vi "HFRR ADV v037.vi"() -> ()   [LabVIEW 2025] (continued)
        n1323 = Not(x=w1614) -> (.not. x?=w1612:bool)
        n1324 = local write "Stroke"(w1612) -> ()
        n1325 = local write "Tab Control 2"(T6."Stroke" ("Tab Control 2")) -> ()
      }
    }
    n1326 = local write "tested by"(w1341) -> ()
    n1327 = case shown="True" w1337 {
      selector: w1337 -> [_ w1617]
      frame False {
      }
      frame True {
        n1328 = Not(x=w1617) -> (.not. x?=w1615:bool)
        n1329 = local write "Humidity"(w1615) -> ()
        n1330 = local write "Tab Control 2"(T6."Humidity" ("Tab Control 2")) -> ()
      }
    }
    n1331 = case shown="\"Calibration\"" "Main Dashboard Buttons" {
      tunnel: [T2."HOME" ("Main Tab") T2."Test Setup" ("Main Tab") T2."Acquire" ("Main Tab") T2."Adv Scar" ("Main Tab") T2."Adv Scar Report" ("Main Tab") T2."Compare Files" ("Main Tab") T2."Calibration" ("Main Tab") T2."About" ("Main Tab") T2."Advance" ("Main Tab")] -> w1320
      frame "Home", Default {
      }
      frame "Test Setup" {
      }
      frame "Dashboard" {
      }
      frame "Imaging" {
      }
      frame "Report" {
      }
      frame "Analysis" {
      }
      frame "Calibration" {
      }
      frame "About" {
      }
      frame "Advance" {
      }
    }
    n1332 = Wait (ms)(milliseconds to wait=u32 100) -> ()  [unwired: 1 out]
    n1333 = local read "Main Tab Display"() -> (w1340:T4)
    n1334 = local write "Main Tab"(w1320) -> ()
    n1335 = case shown="\"Dashboard 3\"" w1340 {
      frame "Dashboard 1", Default {
        n1336 = property on="Reset Graph" class="Bool (strict)"("Visible"=FALSE) -> ()  [unwired: 2 in, 2 out]
      }
      frame "Dashboard 2" {
        n1337 = property on="Reset Graph" class="Bool (strict)"("Visible"=TRUE) -> ()  [unwired: 2 in, 2 out]
      }
      frame "Dashboard 3" {
        n1338 = property on="Reset Graph" class="Bool (strict)"("Visible"=TRUE) -> ()  [unwired: 2 in, 2 out]
      }
    }
    n1339 = local read "SCAR MEASURMENT"() -> (w1328:enum32{"Auto Scar", "Manual Scar"})
    n1340 = local read "Humidity"() -> (w1342:bool)
    n1341 = local read "Cap Live Image"() -> (w1325:bool)
    n1342 = local read "Sample Temperature"() -> (w1335:bool)
    n1343 = local read "Air Temp vs Humidity"() -> (w1333:bool)
    n1344 = local read "Frequency"() -> (w1334:bool)
    n1345 = case shown="False" w1342 {
      frame False {
        n1346 = local write "Humidity On Command"(TRUE ("Humidity On Command")) -> ()
        n1347 = case shown="True" "Humidity Off Command" {
          selector: "Humidity Off Command" -> [_ w1630]
          frame False {
          }
          frame True {
            n1348 = stacked-sequence {
              frame #0 {
                n1349 = local read "WriteHumidity"() -> (w1632:string[])
                n1350 = Insert Into Array(array=w1632, new element="R;1" ("new element/subarray")) -> (w1631:string[])  [unwired: 1 in]
                n1351 = local write "WriteHumidity"(w1631) -> ()
              }
              frame #1 {
                n1352 = Wait (ms)(milliseconds to wait=u32 500) -> ()  [unwired: 1 out]
              }
              frame #2 {
                n1353 = local read "WriteHumidity"() -> (w1636:string[])
                n1354 = local read "EVENT LOG"() -> (w1640:string)
                n1355 = call "Event Log.vi"("Content"="Humidity Control Off" ("string"), "EVENT LOG"=w1640) -> ("EVENT LOG"=w1641:string)  [unwired: 8 in, 1 out]
                n1356 = local write "EVENT LOG"(w1641) -> ()
                n1357 = Insert Into Array(array=w1636, new element="R;1" ("new element/subarray")) -> (w1637:string[])  [unwired: 1 in]
                n1358 = local write "WriteHumidity"(w1637) -> ()
                n1359 = local write "Humidity"(TRUE ("Humidity")) -> ()
              }
            }
            n1360 = Not(x=w1630) -> (.not. x?=w1629:bool)
            n1361 = local write "Humidity Off Command"(w1629) -> ()
          }
        }
      }
      frame True {
        n1362 = local write "Humidity Off Command"(TRUE ("Humidity Off Command")) -> ()
        n1363 = case shown="False" "Humidity On Command" {
          selector: "Humidity On Command" -> [_ w1645]
          frame False {
          }
          frame True {
            n1364 = stacked-sequence {
              frame #0 {
                n1365 = local read "Set Rh"() -> (w1651:dbl)
                n1366 = local read "WriteHumidity"() -> (w1647:string[])
                n1367 = Number To Fractional String(number=w1651, precision (6)=i16 2) -> (F-format string=w1652:string)  [unwired: 2 in]
                n1368 = Concatenate Strings("M;" ("new element/subarray"), w1652) -> (w1650:string)
                n1369 = Insert Into Array(array=w1647, new element=w1650) -> (w1646:string[])  [unwired: 1 in]
                n1370 = local write "WriteHumidity"(w1646) -> ()
              }
              frame #1 {
                n1371 = Wait (ms)(milliseconds to wait=u32 500) -> ()  [unwired: 1 out]
              }
              frame #2 {
                n1372 = local read "WriteHumidity"() -> (w1655:string[])
                n1373 = local read "Set Rh"() -> (w1659:dbl)
                n1374 = Number To Fractional String(number=w1659, precision (6)=i16 2) -> (F-format string=w1660:string)  [unwired: 2 in]
                n1375 = Concatenate Strings("M;" ("new element/subarray"), w1660) -> (w1658:string)
                n1376 = Insert Into Array(array=w1655, new element=w1658) -> (w1654:string[])  [unwired: 1 in]
                n1377 = local write "WriteHumidity"(w1654) -> ()
              }
              frame #3 {
                n1378 = Wait (ms)(milliseconds to wait=u32 500) -> ()  [unwired: 1 out]
              }
              frame #4 {
                (unwired) "% RH" ("string")
                (unwired) i16 2 ("precision (6)")
                (unwired) "M;" ("new element/subarray")
                n1379 = local read "Set Rh"() -> (w1669:dbl)
                n1380 = local read "WriteHumidity"() -> (w1662:string[])
                n1381 = Number To Fractional String(number=w1669, precision (6)=i16 2) -> (F-format string=w1666:string)  [unwired: 2 in]
                n1382 = Concatenate Strings("M;" ("new element/subarray"), w1666) -> (w1670:string)
                n1383 = Concatenate Strings("Humidity Set to : " ("string"), w1666, "% RH" ("string")) -> (w1664:string)
                n1384 = Insert Into Array(array=w1662, new element=w1670) -> (w1663:string[])  [unwired: 1 in]
                n1385 = disable-structure shown="Enabled" {
                  frame Enabled {
                    n1386 = local read "EVENT LOG"() -> (w1673:string)
                    n1387 = call "Event Log.vi"("Content"="Humidity Control On", "EVENT LOG"=w1673) -> ("EVENT LOG"=w1674:string)  [unwired: 8 in, 1 out]
                    n1388 = local write "EVENT LOG"(w1674) -> ()
                  }
                  frame Disabled {
                  }
                }
                n1389 = disable-structure shown="Enabled" {
                  disable-tunnel: w1664 -> [_ _]
                  frame Enabled {
                    n1390 = local read "EVENT LOG"() -> (w1676:string)
                    n1391 = call "Event Log.vi"("Content"="Humidity Control On", "EVENT LOG"=w1676) -> ("EVENT LOG"=w1677:string)  [unwired: 8 in, 1 out]
                    n1392 = local write "EVENT LOG"(w1677) -> ()
                  }
                  frame Disabled {
                  }
                }
                n1393 = local write "WriteHumidity"(w1663) -> ()
              }
            }
            n1394 = Not(x=w1645) -> (.not. x?=w1644:bool)
            n1395 = local write "Humidity On Command"(w1644) -> ()
          }
        }
      }
    }
    n1396 = Equal?(x=w1328, y=enum32{"Auto Scar", "Manual Scar"}."Auto Scar" ("SCAR MEASURMENT")) -> (x = y?=w1324:bool)
    n1397 = local read "TEST STANDARD"() -> (w1331:T3)
    n1398 = And(x=w1325, y=w1324) -> (x .and. y?=w1326:bool)
    n1399 = case shown="True" w1326 {
      selector: w1326 -> [_ w1429]
      tunnel: errorcluster {"status"=FALSE, "code"=0, "source"=""} ("error in (no error) 3") -> [_ w1430]
      frame False {
      }
      frame True {
        n1400 = stacked-sequence {
          tunnel: w1430 -> [_ _ _ _ _ _ _ w1478]
          tunnel: w1429 -> [_ _ _ _ _ w1459 _ _]
          frame #0 {
            n1401 = call "CAMERA LIVE FEED FGV.vi"("Enum - Menu"=CAMERA_LIVE_FEED_ENUM."CAMERA MINIMIZE") -> ()  [unwired: 9 in, 2 out]
          }
          frame #1 {
            n1402 = property on="Auto Scar Check  2" class="Clust (strict)"("Visible"=TRUE) -> ()  [unwired: 2 in, 2 out]
          }
          frame #2 {
            n1403 = String To Path(string="C:\\LAB-IQ\\Image Calibrate v01.dcf") -> (path=w1435:path)
            n1404 = Open/Create/Replace File ("Open File")(file path (use dialog)=w1435) -> (refnum out=w1436:refnum<file>)  [unwired: 5 in, 2 out]
            n1405 = for {
              N: 4 -> [_]
              tunnel: w1436 -> [w1442]
              i -> [w1438]
              n1406 = Read from Text File ("Read File")(file (use dialog)=w1442) -> (text=w1443:string)  [unwired: 3 in, 3 out]
              n1407 = String Subset(string=w1443, offset (0)=6, length (rest)=10 ("length (rest)")) -> (substring=w1439:string)
              n1408 = Fract/Exp String To Number(string=w1439) -> (number=w1437:dbl)  [unwired: 3 in, 1 out]
              n1409 = case shown="0" w1438 {
                tunnel: w1437 -> [w1444 w1445 _ w1446 _]
                frame 0 {
                  "5x Gain" <- w1444
                }
                frame 1 {
                  "10x Gain" <- w1445
                }
                frame 2 {
                }
                frame 3 {
                  "100x gain" <- w1446
                }
                frame 4, Default {
                }
              }
            }
          }
          frame #3 {
            n1410 = local read "FILE 3"() -> (w1452:string)
            n1411 = call <vilib>:"Trim Whitespace.vi"("string"="C:\\LAB-IQ\\images\\") -> ("trimmed string"=w1454:string)  [unwired: 1 in]
            n1412 = String To Path(string=w1454) -> (path=w1453:path)
            n1413 = Concatenate Strings(w1452, ".png" ("string")) -> (w1451:string)
            n1414 = Build Path(base path=w1453, name or relative path=w1451) -> (appended path=w1449:path)
            "Image path" <- w1449
            n1415 = Path To String(path=w1449) -> (string=w1448:string)
            n1416 = call "CAMERA LIVE FEED FGV.vi"("Enum - Menu"=CAMERA_LIVE_FEED_ENUM."CAMERA SAVE", "Image Path"=w1448) -> ()  [unwired: 8 in, 2 out]
          }
          frame #4 {
            n1417 = One Button Dialog(message="Image saved successfully") -> ()  [unwired: 1 in, 1 out]
          }
          frame #5 {
            n1418 = local read "TEST STANDARD"() -> (w1458:T3)
            n1419 = local read "Magnification len live scar"() -> (w1470:string)
            n1420 = Not(x=w1459) -> (.not. x?=w1460:bool)
            n1421 = local write "Cap Live Image"(w1460) -> ()
            n1422 = case shown="\"ISO 12156\"" w1458 {
              tunnel: ["ASTM D6079" "ISO 12156"] -> w1457
              frame "ASTM D6079", Default {
              }
              frame "ISO 12156" {
              }
            }
            n1423 = case shown="\"5x\", Default" w1470 {
              tunnel: [w1473 w1474] -> w1469
              frame "5x", Default {
                n1424 = local read "5x Gain"() -> (w1473:dbl)
              }
              frame "10x" {
                # "5x"
                n1425 = local read "10x Gain"() -> (w1474:dbl)
              }
            }
            n1426 = local read "Image path"() -> (w1468:path)
            n1427 = local read "FILE 3"() -> (w1461:string)
            n1428 = call "EDGE DETCTION.vi"("GAIN VALUE"=w1469, "Image Path"=w1468) -> ("error out"=w1467:errorcluster, "return value"=w1466:cluster{string, string, dbl, dbl, dbl})  [unwired: 8 in]
            n1429 = Bundle By Name(cluster=T27 {"File Name"="", "Test Method"="", "Operator"="", "Fuel Description"="", "Date and time"=""} ("Main Ref"), "File Name"=w1461, "Test Method"=w1457) -> (w1462:T27)
            n1430 = call "duf file read.vi"("error in (no error)"=w1467, "Main Ref"=w1462) -> ("error out"=w1465:errorcluster, "Main Ref 2"=w1463:T27)  [unwired: 8 in]
            n1431 = call "EDGE DETECTION REPORT.vi"("error in (no error)"=w1465, "return value 2"=w1466, "Main Ref"=w1463) -> ()  [unwired: 8 in, 1 out]
          }
          frame #6 {
            n1432 = property on="Auto Scar Check  2" class="Clust (strict)"("Visible"=FALSE) -> ()  [unwired: 2 in, 2 out]
          }
          frame #7 {
            n1433 = call "CAMERA LIVE FEED FGV.vi"("Enum - Menu"=CAMERA_LIVE_FEED_ENUM."CAMERA MINIMIZE", "error in (no error)"=w1478) -> ()  [unwired: 8 in, 2 out]
            n1434 = local write "Main Dashboard Buttons"(T1."Home" ("Main Dashboard Buttons")) -> ()
            n1435 = local write "Main Tab"(T2."HOME" ("Main Tab")) -> ()
          }
        }
      }
    }
    n1436 = local read "Heater Button"() -> (w1332:bool)
    n1437 = case shown="True" w1334 {
      selector: w1334 -> [_ w1608]
      frame False {
      }
      frame True {
        n1438 = Not(x=w1608) -> (.not. x?=w1606:bool)
        n1439 = local write "Frequency"(w1606) -> ()
        n1440 = local write "Tab Control 2"(T6."Frequency" ("Tab Control 2")) -> ()
      }
    }
    n1441 = case shown="True" w1333 {
      selector: w1333 -> [_ w1605]
      frame False {
      }
      frame True {
        n1442 = Not(x=w1605) -> (.not. x?=w1603:bool)
        n1443 = local write "Air Temp vs Humidity"(w1603) -> ()
        n1444 = local write "Tab Control 2"(T6."Air Temp vs Rh" ("Tab Control 2")) -> ()
      }
    }
    n1445 = case shown="True" w1335 {
      selector: w1335 -> [_ w1611]
      frame False {
      }
      frame True {
        n1446 = Not(x=w1611) -> (.not. x?=w1609:bool)
        n1447 = local write "Sample Temperature"(w1609) -> ()
        n1448 = local write "Tab Control 2"(T6."Sample Temperature" ("Tab Control 2")) -> ()
      }
    }
    n1449 = case shown="\"Custom\"" w1331 {
      frame "ASTM D6079", Default {
        w1584 = "ASTM D6079 TEST CONDITIONS" ("Standard 2")
        n1450 = local write "Standard 2"(w1584) -> ()
        n1451 = local write "Standard"(w1584) -> ()
      }
      frame "ISO 12156" {
        w1585 = "ISO 12156 TEST CONDITIONS" ("Standard 2")
        n1452 = local write "Standard 2"(w1585) -> ()
        n1453 = local write "Standard"(w1585) -> ()
      }
      frame "CEC F-096-A-06" {
        w1586 = "CEC F-096-A-06 TEST CONDITIONS" ("Standard 2")
        n1454 = local write "Standard 2"(w1586) -> ()
        n1455 = local write "Standard"(w1586) -> ()
      }
      frame "Custom" {
        w1587 = "CUSTOM TEST CONDITIONS" ("Standard 2")
        n1456 = local write "Standard 2"(w1587) -> ()
        n1457 = local write "Standard"(w1587) -> ()
      }
    }
    n1458 = case shown="True" w1332 {
      frame False {
        n1459 = local write "Temperature On Command"(TRUE ("Temperature On Command")) -> ()
        n1460 = case shown="True" "Temperature Off Command" {
          selector: "Temperature Off Command" -> [_ w1591]
          frame False {
          }
          frame True {
            n1461 = Not(x=w1591) -> (.not. x?=w1590:bool)
            n1462 = local read "EVENT LOG"() -> (w1594:string)
            n1463 = local write "Temperature Off Command"(w1590) -> ()
            n1464 = call "Event Log.vi"("Content"="Heater Off", "EVENT LOG"=w1594) -> ("EVENT LOG"=w1593:string)  [unwired: 8 in, 1 out]
            n1465 = local write "EVENT LOG"(w1593) -> ()
          }
        }
      }
      frame True {
        n1466 = local write "Temperature Off Command"(TRUE ("Temperature Off Command")) -> ()
        n1467 = case shown="True" "Temperature On Command" {
          selector: "Temperature On Command" -> [_ w1598]
          frame False {
          }
          frame True {
            n1468 = Not(x=w1598) -> (.not. x?=w1597:bool)
            n1469 = local write "Temperature On Command"(w1597) -> ()
            n1470 = disable-structure shown="Enabled" {
              disable-tunnel: "Heater On" -> [w1600 _]
              frame Enabled {
                n1471 = local read "EVENT LOG"() -> (w1601:string)
                n1472 = call "Event Log.vi"("Content"=w1600, "EVENT LOG"=w1601) -> ("EVENT LOG"=w1602:string)  [unwired: 8 in, 1 out]
                n1473 = local write "EVENT LOG"(w1602) -> ()
              }
              frame Disabled {
              }
            }
          }
        }
      }
    }
    n1474 = local read "Main Tab"() -> (w1323:T2)
    n1475 = case shown="\"About\"" w1323 {
      frame "HOME", Default {
        w1365 = T19."Enabled" ("Disabled")
        n1476 = local read "Service Password enable"() -> (w1367:bool)
        n1477 = property on="Imaging" class="Bool (strict)"("DisabledEnum"=w1365) -> ()  [unwired: 2 in, 2 out]
        n1478 = property on="Dashboard" class="Bool (strict)"("DisabledEnum"=w1365) -> ()  [unwired: 2 in, 2 out]
        n1479 = property on="Test Setup" class="Bool (strict)"("DisabledEnum"=w1365) -> ()  [unwired: 2 in, 2 out]
        n1480 = property on="Analysis" class="Bool (strict)"("DisabledEnum"=w1365) -> ()  [unwired: 2 in, 2 out]
        n1481 = property on="Home" class="Bool (strict)"("DisabledEnum"=w1365) -> ()  [unwired: 2 in, 2 out]
        n1482 = property on="Report" class="Bool (strict)"("DisabledEnum"=w1365) -> ()  [unwired: 2 in, 2 out]
        n1483 = property on="Main Dashboard Buttons" class="RadioBtnsControl (strict)"("DisabledEnum"=w1365) -> ()  [unwired: 2 in, 2 out]
        n1484 = property on="Calibration" class="Bool (strict)"("DisabledEnum"=w1365) -> ()  [unwired: 2 in, 2 out]
        n1485 = case shown="True" w1367 {
          tunnel: [T19."Disabled" ("Disabled") T19."Enabled" ("Disabled")] -> w1366
          frame False {
          }
          frame True {
          }
        }
        n1486 = property on="About" class="Bool (strict)"("DisabledEnum"=w1366) -> ()  [unwired: 2 in, 2 out]
      }
      frame "Test Setup" {
        w1372 = T19."Enabled" ("Disabled")
        n1487 = local read "Service Password enable"() -> (w1371:bool)
        n1488 = property on="Dashboard" class="Bool (strict)"("DisabledEnum"=T19."Disabled" ("Disabled")) -> ()  [unwired: 2 in, 2 out]
        n1489 = property on="Imaging" class="Bool (strict)"("DisabledEnum"=w1372) -> ()  [unwired: 2 in, 2 out]
        n1490 = property on="Analysis" class="Bool (strict)"("DisabledEnum"=w1372) -> ()  [unwired: 2 in, 2 out]
        n1491 = property on="Home" class="Bool (strict)"("DisabledEnum"=w1372) -> ()  [unwired: 2 in, 2 out]
        n1492 = property on="Report" class="Bool (strict)"("DisabledEnum"=w1372) -> ()  [unwired: 2 in, 2 out]
        n1493 = property on="Test Setup" class="Bool (strict)"("DisabledEnum"=w1372) -> ()  [unwired: 2 in, 2 out]
        n1494 = case shown="True" w1371 {
          tunnel: [T19."Disabled" ("Disabled") T19."Enabled" ("Disabled")] -> w1370
          frame False {
          }
          frame True {
          }
        }
        n1495 = property on="About" class="Bool (strict)"("DisabledEnum"=w1370) -> ()  [unwired: 2 in, 2 out]
      }
      frame "Adv Scar" {
        w1379 = T19."Enabled" ("Disabled")
        n1496 = property on="Dashboard" class="Bool (strict)"("DisabledEnum"=T19."Disabled" ("Disabled")) -> ()  [unwired: 2 in, 2 out]
        n1497 = property on="Imaging" class="Bool (strict)"("DisabledEnum"=w1379) -> ()  [unwired: 2 in, 2 out]
        n1498 = property on="Analysis" class="Bool (strict)"("DisabledEnum"=w1379) -> ()  [unwired: 2 in, 2 out]
        n1499 = property on="Home" class="Bool (strict)"("DisabledEnum"=w1379) -> ()  [unwired: 2 in, 2 out]
        n1500 = property on="Report" class="Bool (strict)"("DisabledEnum"=w1379) -> ()  [unwired: 2 in, 2 out]
        n1501 = property on="Test Setup" class="Bool (strict)"("DisabledEnum"=w1379) -> ()  [unwired: 2 in, 2 out]
        n1502 = local read "Service Password enable"() -> (w1377:bool)
        n1503 = case shown="True" w1377 {
          tunnel: [T19."Disabled" ("Disabled") T19."Enabled" ("Disabled")] -> w1376
          frame False {
          }
          frame True {
          }
        }
        n1504 = property on="About" class="Bool (strict)"("DisabledEnum"=w1376) -> ()  [unwired: 2 in, 2 out]
      }
      frame "Calibration" {
        w1382 = T19."Enabled" ("Disabled")
        n1505 = property on="Dashboard" class="Bool (strict)"("DisabledEnum"=T19."Disabled" ("Disabled")) -> ()  [unwired: 2 in, 2 out]
        n1506 = property on="Imaging" class="Bool (strict)"("DisabledEnum"=w1382) -> ()  [unwired: 2 in, 2 out]
        n1507 = property on="Analysis" class="Bool (strict)"("DisabledEnum"=w1382) -> ()  [unwired: 2 in, 2 out]
        n1508 = property on="Home" class="Bool (strict)"("DisabledEnum"=w1382) -> ()  [unwired: 2 in, 2 out]
        n1509 = property on="Report" class="Bool (strict)"("DisabledEnum"=w1382) -> ()  [unwired: 2 in, 2 out]
        n1510 = property on="Test Setup" class="Bool (strict)"("DisabledEnum"=w1382) -> ()  [unwired: 2 in, 2 out]
        n1511 = local read "Service Password enable"() -> (w1384:bool)
        n1512 = property on="Calibration" class="Bool (strict)"("DisabledEnum"=w1382) -> ()  [unwired: 2 in, 2 out]
        n1513 = case shown="True" w1384 {
          tunnel: [T19."Disabled" ("Disabled") T19."Enabled" ("Disabled")] -> w1383
          frame False {
          }
          frame True {
          }
        }
        n1514 = property on="About" class="Bool (strict)"("DisabledEnum"=w1383) -> ()  [unwired: 2 in, 2 out]
      }
      frame "Adv Scar Report" {
        w1390 = T19."Enabled" ("Disabled")
        n1515 = property on="Dashboard" class="Bool (strict)"("DisabledEnum"=T19."Disabled" ("Disabled")) -> ()  [unwired: 2 in, 2 out]
        n1516 = property on="Imaging" class="Bool (strict)"("DisabledEnum"=w1390) -> ()  [unwired: 2 in, 2 out]
        n1517 = property on="Analysis" class="Bool (strict)"("DisabledEnum"=w1390) -> ()  [unwired: 2 in, 2 out]
        n1518 = property on="Home" class="Bool (strict)"("DisabledEnum"=w1390) -> ()  [unwired: 2 in, 2 out]
        n1519 = property on="Report" class="Bool (strict)"("DisabledEnum"=w1390) -> ()  [unwired: 2 in, 2 out]
        n1520 = property on="Test Setup" class="Bool (strict)"("DisabledEnum"=w1390) -> ()  [unwired: 2 in, 2 out]
        n1521 = local read "Service Password enable"() -> (w1389:bool)
        n1522 = case shown="True" w1389 {
          tunnel: [T19."Disabled" ("Disabled") T19."Enabled" ("Disabled")] -> w1388
          frame False {
          }
          frame True {
          }
        }
        n1523 = property on="About" class="Bool (strict)"("DisabledEnum"=w1388) -> ()  [unwired: 2 in, 2 out]
      }
      frame "Compare Files" {
        w1396 = T19."Enabled" ("Disabled")
        n1524 = local read "Service Password enable"() -> (w1395:bool)
        n1525 = property on="Dashboard" class="Bool (strict)"("DisabledEnum"=T19."Disabled" ("Disabled")) -> ()  [unwired: 2 in, 2 out]
        n1526 = property on="Imaging" class="Bool (strict)"("DisabledEnum"=w1396) -> ()  [unwired: 2 in, 2 out]
        n1527 = property on="Analysis" class="Bool (strict)"("DisabledEnum"=w1396) -> ()  [unwired: 2 in, 2 out]
        n1528 = property on="Home" class="Bool (strict)"("DisabledEnum"=w1396) -> ()  [unwired: 2 in, 2 out]
        n1529 = property on="Report" class="Bool (strict)"("DisabledEnum"=w1396) -> ()  [unwired: 2 in, 2 out]
        n1530 = property on="Test Setup" class="Bool (strict)"("DisabledEnum"=w1396) -> ()  [unwired: 2 in, 2 out]
        n1531 = case shown="True" w1395 {
          tunnel: [T19."Disabled" ("Disabled") T19."Enabled" ("Disabled")] -> w1394
          frame False {
          }
          frame True {
          }
        }
        n1532 = property on="About" class="Bool (strict)"("DisabledEnum"=w1394) -> ()  [unwired: 2 in, 2 out]
      }
      frame "Acquire" {
        n1533 = local read "Service Password enable"() -> (w1401:bool)
        n1534 = property on="Test Setup" class="Bool (strict)"("DisabledEnum"=T19."Disabled" ("Disabled")) -> ()  [unwired: 2 in, 2 out]
        n1535 = local read "Auto Start Test"() -> (w1403:bool)
        n1536 = local read "RUN"() -> (w1405:bool)
        n1537 = case shown="True" w1401 {
          tunnel: [T19."Disabled" ("Disabled") T19."Enabled" ("Disabled")] -> w1402
          frame False {
          }
          frame True {
          }
        }
        n1538 = Or(x=w1405, y=w1403) -> (x .or. y?=w1404:bool)
        n1539 = case shown="True" w1404 {
          tunnel: [T19."Enabled" ("Disabled") T19."Disabled" ("Disabled")] -> w1400
          frame False {
          }
          frame True {
          }
        }
        n1540 = property on="About" class="Bool (strict)"("DisabledEnum"=w1402) -> ()  [unwired: 2 in, 2 out]
        n1541 = property on="Imaging" class="Bool (strict)"("DisabledEnum"=w1400) -> ()  [unwired: 2 in, 2 out]
        n1542 = property on="Dashboard" class="Bool (strict)"("DisabledEnum"=w1400) -> ()  [unwired: 2 in, 2 out]
        n1543 = property on="Analysis" class="Bool (strict)"("DisabledEnum"=w1400) -> ()  [unwired: 2 in, 2 out]
        n1544 = property on="Home" class="Bool (strict)"("DisabledEnum"=w1400) -> ()  [unwired: 2 in, 2 out]
        n1545 = property on="Report" class="Bool (strict)"("DisabledEnum"=w1400) -> ()  [unwired: 2 in, 2 out]
        n1546 = property on="Calibration" class="Bool (strict)"("DisabledEnum"=w1400) -> ()  [unwired: 2 in, 2 out]
      }
      frame "About" {
        n1547 = local read "FILE"() -> (w1419:string)
        n1548 = local read "TEST FILE NAM,E SAVED"() -> (w1412:bool)
        n1549 = call <vilib>:"Trim Whitespace.vi"("string"=w1419) -> ("trimmed string"=w1418:string)  [unwired: 1 in]
        n1550 = local read "Auto Start Test"() -> (w1422:bool)
        n1551 = String Length(string=w1418) -> (length=w1417:i32)
        n1552 = Greater?(x=w1417, y=1) -> (0:w1414:bool)
        n1553 = And(x=w1414, y=w1412) -> (x .and. y?=w1413:bool)
        n1554 = local read "RUN"() -> (w1424:bool)
        n1555 = case shown="True" w1413 {
          tunnel: [T19."Disabled" ("Disabled") T19."Enabled" ("Disabled")] -> w1415
          frame False {
          }
          frame True {
          }
        }
        n1556 = Or(x=w1424, y=w1422) -> (x .or. y?=w1423:bool)
        n1557 = property on="About" class="Bool (strict)"("DisabledEnum"=T19."Enabled" ("Disabled")) -> ()  [unwired: 2 in, 2 out]
        n1558 = case shown="False" w1423 {
          tunnel: [T19."Enabled" ("Disabled") T19."Disabled" ("Disabled")] -> w1421
          frame False {
          }
          frame True {
          }
        }
        n1559 = property on="Dashboard" class="Bool (strict)"("DisabledEnum"=w1415) -> ()  [unwired: 2 in, 2 out]
        n1560 = property on="Test Setup" class="Bool (strict)"("DisabledEnum"=T19."Disabled" ("Disabled")) -> ()  [unwired: 2 in, 2 out]
        n1561 = property on="Imaging" class="Bool (strict)"("DisabledEnum"=w1421) -> ()  [unwired: 2 in, 2 out]
        n1562 = property on="Analysis" class="Bool (strict)"("DisabledEnum"=w1421) -> ()  [unwired: 2 in, 2 out]
        n1563 = property on="Home" class="Bool (strict)"("DisabledEnum"=w1421) -> ()  [unwired: 2 in, 2 out]
        n1564 = property on="Report" class="Bool (strict)"("DisabledEnum"=w1421) -> ()  [unwired: 2 in, 2 out]
      }
    }
    n1565 = local read "Quit"() -> (w1349:bool)
    "Single" <- "Single - Graph"
  }
  n1566 = disable-structure shown="Disabled" {
    disable-tunnel: [w1702 _] -> w42
    disable-tunnel: _ -> [w1701 _]
    frame Disabled {
      n1567 = while {
        tunnel: w1701 -> [_]
        tunnel: [w1703] -> w1702
        tunnel: [w1704] -> _
        i -> [w1704]
        stop <- w1703 stop-if-true
        w1720 = u16 10 items=["1.0"=10, "1.5"=15, "2.0"=20] ("stop bits (10: 1 bit)")
        n1568 = Wait (ms)(milliseconds to wait=u32 10) -> ()  [unwired: 1 out]
        n1569 = call-poly "VISA Configure Serial Port"("VISA resource name"=refnum<visa-resource-name> "ASRL1::INSTR" ("COM PORT"), "timeout (10sec)"=u32 10, "baud rate (9600)"=u32 57600, "data bits (8)"=u16 8, "stop bits (10: 1 bit)"=w1720) -> ("VISA resource name out"=w1706:refnum<visa-resource-name>, "error out"=w1715:errorcluster)  [unwired: 9 in]
        n1570 = VISA Read(VISA resource name=w1706, byte count=u32 2 ("byte count (0)")) -> (read buffer=w1714:string)  [unwired: 1 in, 3 out]
        n1571 = String Subset(string=w1714, offset (0)=0, length (rest)=2 ("length (rest)")) -> (substring=w1713:string)
        n1572 = Match Pattern(string=w1713, regular expression="<>") -> (offset past match=w1710:i32)  [unwired: 1 in, 3 out]
        n1573 = Greater Or Equal?(x=w1710, y=0) -> (x >= y?=w1705:bool)
        n1574 = case shown="True" w1705 {
          tunnel: w1706 -> [_ w1724]
          tunnel: w1715 -> [_ w1723]
          frame False {
          }
          frame True {
            n1575 = VISA Read(VISA resource name=w1724, byte count=u32 32 ("byte count (0)"), error in (no error)=w1723) -> (read buffer=w1722:string)  [unwired: 3 out]
            n1576 = String Subset(string=w1722, offset (0)=0, length (rest)=8 ("length (rest)")) -> (substring=w1726:string)
            n1577 = String Subset(string=w1722, offset (0)=8, length (rest)=8 ("length (rest)")) -> (substring=w1727:string)
            n1578 = Decimal String To Number(string=w1727) -> (number=w1734:i32)  [unwired: 2 in, 1 out]
            n1579 = Decimal String To Number(string=w1726) -> (number=w1730:i32)  [unwired: 2 in, 1 out]
            n1580 = Divide(x=w1734, y=10000) -> ()  [unwired: 1 out]
            n1581 = Divide(x=w1730, y=1000000) -> ()  [unwired: 1 out]
          }
        }
        n1582 = local read "Quit"() -> (w1703:bool)
      }
    }
    frame Enabled {
    }
  }
  n1583 = Tick Count (ms)() -> (millisecond timer value=w4:u32)
  n1584 = while {
    shift-right: [w1780] -> _
    shift-left: w6 -> [w1784]
    shift-right: [w1779] -> _
    shift-left: w5 -> [w1783]
    shift-right: [w1778] -> _
    shift-left: w6 -> [w1782]
    shift-right: [w1777] -> _
    shift-left: w5 -> [w1781]
    shift-right: [w1775] -> _
    shift-left: w4 -> [w1776]
    shift-right: [w1772] -> _
    shift-left: w3 -> [w1773]
    shift-right: [w1771] -> _
    shift-left: w3 -> [w1774]
    shift-right: [w1764] -> _
    shift-left: w3 -> [w1770]
    shift-right: [w1763] -> _
    shift-left: w3 -> [w1769]
    shift-right: [w1762] -> _
    shift-left: w3 -> [w1768]
    shift-right: [w1761] -> _
    shift-left: w3 -> [w1767]
    shift-right: [w1760] -> _
    shift-left: w3 -> [w1766]
    shift-right: [w1759] -> _
    shift-left: w3 -> [w1765]
    shift-right: [w1758] -> _
    shift-left: w3 -> [w1752]
    shift-right: [w1757] -> _
    shift-left: w3 -> [w1751]
    shift-right: [w1756] -> _
    shift-left: w3 -> [w1750]
    shift-right: [w1755] -> _
    shift-left: w3 -> [w1749]
    shift-right: [w1754] -> _
    shift-left: w3 -> [w1748]
    shift-right: [w1753] -> _
    shift-left: w3 -> [w1747]
    shift-right: [w1738] -> _
    shift-left: w3 -> [w1741]
    shift-right: [w1737] -> _
    shift-left: w3 -> [w1740]
    shift-right: [w1736] -> _
    shift-left: w3 -> [w1739]
    stop <- w1786 stop-if-true
    n1585 = local read "Read UNO"() -> (w1745:string)
    n1586 = local read "Error  2"() -> (w1785:errorcluster)
    n1587 = String Length(string=w1745) -> (length=w1744:i32)
    n1588 = call <vilib>:"Trim Whitespace.vi"("string"=w1745) -> ("trimmed string"=w1746:string)  [unwired: 1 in]
    n1589 = Greater Or Equal?(x=w1744, y=23) -> (x >= y?=w1742:bool)
    n1590 = case shown="No Error" w1785 {
      tunnel: w1784 -> [w1832 w1928]
      tunnel: w1783 -> [w1831 w1927]
      tunnel: w1782 -> [w1830 w1926]
      tunnel: w1781 -> [w1829 w1925]
      tunnel: [w1828 w1928] -> w1780
      tunnel: [w1827 w1927] -> w1779
      tunnel: [w1826 w1926] -> w1778
      tunnel: [w1825 w1925] -> w1777
      tunnel: w1776 -> [w1824 w1924]
      tunnel: [w1823 w1924] -> w1775
      tunnel: w1773 -> [w1822 w1923]
      tunnel: w1774 -> [w1821 w1922]
      tunnel: [w1820 w1923] -> w1772
      tunnel: [w1819 w1922] -> w1771
      tunnel: w1770 -> [w1818 w1921]
      tunnel: w1769 -> [w1817 w1920]
      tunnel: w1768 -> [w1816 w1919]
      tunnel: w1767 -> [w1815 w1918]
      tunnel: w1766 -> [w1814 w1917]
      tunnel: w1765 -> [w1813 w1916]
      tunnel: [w1812 w1921] -> w1764
      tunnel: [w1811 w1920] -> w1763
      tunnel: [w1810 w1919] -> w1762
      tunnel: [w1809 w1918] -> w1761
      tunnel: [w1808 w1917] -> w1760
      tunnel: [w1807 w1916] -> w1759
      tunnel: w1752 -> [w1806 w1915]
      tunnel: [w1805 w1915] -> w1758
      tunnel: [w1804 w1911] -> w1757
      tunnel: [w1803 w1910] -> w1756
      tunnel: [w1802 w1914] -> w1755
      tunnel: [w1801 w1913] -> w1754
      tunnel: [w1800 w1912] -> w1753
      tunnel: w1751 -> [w1799 w1914]
      tunnel: w1750 -> [w1798 w1913]
      tunnel: w1749 -> [w1797 w1912]
      tunnel: w1748 -> [w1796 w1911]
      tunnel: w1747 -> [w1795 w1910]
      tunnel: w1746 -> [w1794 _]
      tunnel: w1742 -> [w1793 _]
      tunnel: w1741 -> [w1792 w1909]
      tunnel: w1740 -> [w1791 w1908]
      tunnel: w1739 -> [w1790 w1907]
      tunnel: [w1789 w1909] -> w1738
      tunnel: [w1788 w1908] -> w1737
      tunnel: [w1787 w1907] -> w1736
      frame No Error {
        n1591 = case shown="True" w1793 {
          tunnel: w1832 -> [w1848 w1900]
          tunnel: w1831 -> [w1847 w1899]
          tunnel: w1830 -> [w1846 w1898]
          tunnel: w1829 -> [w1845 w1897]
          tunnel: [w1848 w1896] -> w1828
          tunnel: [w1847 w1895] -> w1827
          tunnel: [w1846 w1894] -> w1826
          tunnel: [w1845 w1893] -> w1825
          tunnel: w1824 -> [w1844 w1891]
          tunnel: [w1844 w1890] -> w1823
          tunnel: w1822 -> [w1843 w1889]
          tunnel: w1821 -> [w1842 w1888]
          tunnel: [w1843 w1887] -> w1820
          tunnel: [w1842 w1886] -> w1819
          tunnel: w1818 -> [w1841 w1885]
          tunnel: w1817 -> [w1840 w1884]
          tunnel: w1816 -> [w1839 w1883]
          tunnel: w1815 -> [w1838 w1882]
          tunnel: w1814 -> [w1837 w1881]
          tunnel: w1813 -> [w1836 w1880]
          tunnel: [w1841 w1879] -> w1812
          tunnel: [w1840 w1878] -> w1811
          tunnel: [w1839 w1877] -> w1810
          tunnel: [w1838 w1876] -> w1809
          tunnel: [w1837 w1875] -> w1808
          tunnel: [w1836 w1874] -> w1807
          tunnel: w1806 -> [w1854 w1873]
          tunnel: [w1854 w1872] -> w1805
          tunnel: [w1851 w1871] -> w1804
          tunnel: [w1850 w1870] -> w1803
          tunnel: [w1853 w1869] -> w1802
          tunnel: [w1849 w1868] -> w1801
          tunnel: [w1852 w1867] -> w1800
          tunnel: w1799 -> [w1853 w1866]
          tunnel: w1798 -> [w1852 w1865]
          tunnel: w1797 -> [w1851 w1864]
          tunnel: w1796 -> [w1850 w1863]
          tunnel: w1795 -> [w1849 w1862]
          tunnel: w1794 -> [_ w1861]
          tunnel: w1792 -> [w1835 w1860]
          tunnel: w1791 -> [w1834 w1859]
          tunnel: w1790 -> [w1833 w1858]
          tunnel: [w1835 w1857] -> w1789
          tunnel: [w1834 w1856] -> w1788
          tunnel: [w1833 w1855] -> w1787
          frame False {
          }
          frame True {
            n1592 = Tick Count (ms)() -> (millisecond timer value=w1892:u32)
            n1593 = String To Byte Array(string=w1861) -> (unsigned byte array=w1905:u8[])
            n1594 = Array Size(array=w1905) -> (size(s)=w1904:i32)
            n1595 = formula code="// --- INTERNAL VARIABLE DECLARATIONS ---\nint i = 0;\nint k = 0;\nint start_idx = -1;\nint end_idx = -1;\nint phase = 0;\nint sign0 = 1;\nint sign1 = 1;\nint ch0_val = 0;   \nint ch1_val = 0;   \nfloat ch0_raw = 0.0;\nfloat ch1_raw = 0.0;\nfloat temp0 = 0.0;\nfloat temp1 = 0.0;\nfloat ch0_clean = 0.0;\nfloat ch1_clean = 0.0;\n\nint valid_samples = 0; // FIX: Track if we actually parsed new data this window\nfloat max_allowed_bits = 8388607.0; // FIX: Change this to match your ADC max value\n\n// Temporal intermediate variables for calculation smoothing\nfloat raw_p2p_v = 0.0;\nfloat raw_friction = 0.0;\nfloat raw_cof = 0.0;\n\n// Temporal intermediate variables for Piezo voltage translations\nfloat piezo_min_v = 0.0;\nfloat piezo_max_v = 0.0;\n\n// Initialize output variables to current shift register states right away\nout_LVDT_Min_V = in_LVDT_Min_V;\nout_LVDT_Max_V = in_LVDT_Max_V;\nout_LVDT_P2P_V = in_LVDT_P2P_V;\nout_Piezo_P2P = in_Piezo_P2P;\nout_Friction_N = in_Friction_N;\nout_COF = in_COF;\nwindow_ready = 0;\n\n// --- STEP 1: PARSE EVERY STRING IN THE BYTE ARRAY ---\nif (array_size > 2) {\n    for (i = 0; i < array_size - 1; i++) {\n        if (raw_bytes[i] == 42) { // '*' character detected\n            start_idx = i;\n        }\n        \n        // Match standard delimiter sequence \";&\" or end window character\n        if (raw_bytes[i] == 59 && raw_bytes[i+1] == 38 && start_idx != -1) { \n            end_idx = i;\n            ch0_val = 0;\n            ch1_val = 0;\n            sign0 = 1;\n            sign1 = 1;\n            phase = 0; \n\n            for (k = start_idx + 1; k < end_idx; k++) {\n                if (raw_bytes[k] == 45) { // '-' sign\n                    if (phase == 0) sign0 = -1;\n                    else sign1 = -1;\n                }\n                else if (raw_bytes[k] == 43) { // '+' sign\n                    if (phase == 0) sign0 = 1;\n                    else sign1 = 1;\n                }\n                else if (raw_bytes[k] == 59) { // ';' delimiter\n                    phase = 1; \n                }\n                else if (raw_bytes[k] >= 48 && raw_bytes[k] <= 57) { // Numeric ASCII digits\n                    if (phase == 0) {\n                        ch0_val = (ch0_val * 10) + (raw_bytes[k] - 48);\n                    } else {\n                        ch1_val = (ch1_val * 10) + (raw_bytes[k] - 48);\n                    }\n                }\n            }\n\n            // Implicit type conversion\n            ch0_raw = ch0_val * sign0 * 1.0;\n            ch1_raw = ch1_val * sign1 * 1.0;\n\n            // FIX: Sanity check / Hard-clamping to catch sudden massive ASCII noise spikes\n            if (ch0_raw > max_allowed_bits)  ch0_raw = max_allowed_bits;\n            if (ch0_raw < -max_allowed_bits) ch0_raw = -max_allowed_bits;\n            if (ch1_raw > max_allowed_bits)  ch1_raw = max_allowed_bits;\n            if (ch1_raw < -max_allowed_bits) ch1_raw = -max_allowed_bits;\n\n            // --- STEP 2: 3-SAMPLE MEDIAN FILTER ---\n            m0_2 = m0_1; m0_1 = m0_0; m0_0 = ch0_raw;\n            float s0_0 = m0_0; float s0_1 = m0_1; float s0_2 = m0_2;\n            if (s0_0 > s0_1) { temp0 = s0_0; s0_0 = s0_1; s0_1 = temp0; }\n            if (s0_1 > s0_2) { temp0 = s0_1; s0_1 = s0_2; s0_2 = temp0; }\n            if (s0_0 > s0_1) { temp0 = s0_0; s0_0 = s0_1; s0_1 = temp0; }\n            ch0_clean = s0_1;\n\n            m1_2 = m1_1; m1_1 = m1_0; m1_0 = ch1_raw;\n            float s1_0 = m1_0; float s1_1 = m1_1; float s1_2 = m1_2;\n            if (s1_0 > s1_1) { temp1 = s1_0; s1_0 = s1_1; s1_1 = temp1; }\n            if (s1_1 > s1_2) { temp1 = s1_1; s1_1 = s1_2; s1_2 = temp1; }\n            if (s1_0 > s1_1) { temp1 = s1_0; s1_0 = s1_1; s1_1 = temp1; }\n            ch1_clean = s1_1;\n\n            // --- STEP 3: EXPONENTIAL FILTER (STREAM LEVEL) ---\n            if (ch0_filt == 0.0) ch0_filt = ch0_clean;\n            if (ch1_filt == 0.0) ch1_filt = ch1_clean;\n\n            ch0_filt = ch0_filt + (ch0_clean - ch0_filt) * 0.125;\n            ch1_filt = ch1_filt + (ch1_clean - ch1_filt) * 0.125;\n\n            // --- STEP 4: MIN/MAX WINDOW CONTINUOUS ACCUMULATION ---\n            if (ch0_filt > max_ch0) max_ch0 = ch0_filt;\n            if (ch0_filt < min_ch0) min_ch0 = ch0_filt;\n            if (ch1_filt > max_ch1) max_ch1 = ch1_filt;\n            if (ch1_filt < min_ch1) min_ch1 = ch1_filt;\n\n            valid_samples++; // FIX: Successfully parsed and accumulated a clean point\n            start_idx = -1; \n        }\n    }\n}\n\n// --- STEP 5: WINDOW EVALUATION ENGINE ---\n// FIX: Condition updated to verify that valid samples exist for both channels\nif (((current_time_ms - start_time_ms) >= 50) && (valid_samples > 0) && (min_ch0 < 9000000.0) && (min_ch1 < 9000000.0)) {\n    window_ready = 1;\n\n    // Linear Bit-to-Voltage Transformations (LVDT - Channel 0)\n    out_LVDT_Min_V = (min_ch0 * VREF) / 8388607.0;\n    out_LVDT_Max_V = (max_ch0 * VREF) / 8388607.0;\n    raw_p2p_v = out_LVDT_Max_V - out_LVDT_Min_V;\n\n    // Linear Bit-to-Voltage Transformations (Piezo - Channel 1)\n    piezo_min_v = (min_ch1 * VREF) / 8388607.0;\n    piezo_max_v = (max_ch1 * VREF) / 8388607.0;\n    \n    // Assign Peak-to-Peak Voltage directly to output indicator (Matches Python logic)\n    out_Piezo_P2P = piezo_max_v - piezo_min_v;\n    \n    // Force scaling calculations using Voltage delta * Newtons/Volt Factor\n    raw_friction = out_Piezo_P2P * PIEZO_CAL_FACTOR + 0.44528;\n    raw_cof = raw_friction / NORMAL_FORCE;\n\n    // --- STEP 6: OUTPUT METRIC SMOOTHING (Low-Pass Filter Alpha = 0.05) ---\n    // Seed initial historical metrics if first loop iteration\n    if (hist_LVDT_P2P == 0.0) hist_LVDT_P2P = raw_p2p_v;\n    if (hist_Friction == 0.0) hist_Friction = raw_friction;\n    if (hist_COF == 0.0)      hist_COF = raw_cof;\n\n    // Apply exponential output dampening\n    hist_LVDT_P2P = hist_LVDT_P2P + (raw_p2p_v - hist_LVDT_P2P) * 0.05;\n    hist_Friction = hist_Friction + (raw_friction - hist_Friction) * 0.05; // Note: Can drop to 0.02 for more aggressive damping\n    hist_COF      = hist_COF + (raw_cof - hist_COF) * 0.05;\n\n    // Direct smoothed parameters out to UI Indicators\n    out_LVDT_P2P_V = hist_LVDT_P2P;\n    out_Friction_N = hist_Friction;\n    out_COF        = hist_COF;\n\n    // Reset tracking targets to extreme boundaries safely\n    min_ch0 = 9999999.0;\n    max_ch0 = -9999999.0;\n    min_ch1 = 9999999.0;\n    max_ch1 = -9999999.0;\n\n    valid_samples = 0; // FIX: Reset counter for next time frame\n    start_time_ms = current_time_ms;\n}"("raw_bytes"=w1905, "array_size"=w1904, "VREF"="VREF", "PIEZO_CAL_FACTOR"="PIEZO_CAL_FACTOR", "NORMAL_FORCE"="NORMAL_FORCE", "min_ch0"=w1900, "max_ch0"=w1899, "min_ch1"=w1898, "max_ch1"=w1897, "current_time_ms"=w1892, "start_time_ms"=w1891, "ch0_filt"=w1889, "ch1_filt"=w1888, "m0_0"=w1885, "m0_1"=w1884, "m0_2"=w1883, "m1_0"=w1882, "m1_1"=w1881, "m1_2"=w1880, "in_LVDT_Min_V"=w1873, "in_LVDT_Max_V"=w1866, "in_LVDT_P2P_V"=w1865, "in_Piezo_P2P"=w1864, "in_Friction_N"=w1863, "in_COF"=w1862, "hist_LVDT_P2P"=w1860, "hist_Friction"=w1859, "hist_COF"=w1858) -> ("window_ready"=→"Valid_data":dbl, "out_LVDT_Min_V"=w1872:dbl, "out_LVDT_Max_V"=w1871:dbl, "out_LVDT_P2P_V"=w1870:dbl, "out_Piezo_P2P"=w1869:dbl, "out_Friction_N"=w1868:dbl, "out_COF"=w1867:dbl, "min_ch0"=w1896:dbl, "max_ch0"=w1895:dbl, "min_ch1"=w1894:dbl, "max_ch1"=w1893:dbl, "start_time_ms"=w1890:u32, "ch0_filt"=w1887:dbl, "ch1_filt"=w1886:dbl, "m0_0"=w1879:dbl, "m0_1"=w1878:dbl, "m0_2"=w1877:dbl, "m1_0"=w1876:dbl, "m1_1"=w1875:dbl, "m1_2"=w1874:dbl, "hist_LVDT_P2P"=w1857:dbl, "hist_Friction"=w1856:dbl, "hist_COF"=w1855:dbl)
            "LVDT MIN" <- w1872
            "LVDT MAX" <- w1871
            "LVDT Peak" <- w1870
            "pizo raw" <- w1869
            "cof" <- w1867
            "Frictioin Force Raw" <- w1868
          }
        }
      }
      frame Error {
      }
    }
    n1596 = local read "Quit"() -> (w1786:bool)
  }
  n1597 = disable-structure shown="Disabled" {
    disable-tunnel: errorcluster {"status"=TRUE, "code"=0, "source"="Init"} ("error IO") -> [w1931 _]
    disable-tunnel: [w1929 _] -> w45
    frame Disabled {
      n1598 = while {
        shift-right: [w1947] -> w1933
        shift-left: _ -> [w1938]
        shift-right: [w1946] -> w1932
        shift-left: w1931 -> [w1940]
        tunnel: [w1935] -> w1929
        tunnel: [w1945] -> _
        i -> [w1945]
        stop <- w1935 stop-if-true
        n1599 = local read "Port 1a"() -> (w1941:bool)
        n1600 = local read "Port 3"() -> (w1942:bool)
        n1601 = local read "Com Port 1"() -> (w1939:refnum<visa-resource-name>)
        n1602 = Or(x=w1942, y=w1941) -> (x .or. y?=w1944:bool)
        n1603 = Unbundle(w1940) -> ("status"=→"Port 3":bool)  [unwired: 2 out]
        n1604 = Not Equal?(x=w1939, y=w1938) -> (x != y?=w1936:bool)
        n1605 = case shown="True" w1944 {
          frame False {
            w1950 = TRUE ("Visible")
            n1606 = property on="Port 1a" class="Bool (strict)"("Visible"=w1950) -> ()  [unwired: 2 in, 2 out]
            n1607 = property on="Port 3" class="Bool (strict)"("Visible"=w1950) -> ()  [unwired: 2 in, 2 out]
          }
          frame True {
            w1951 = TRUE ("Visible")
            n1608 = property on="Port 1a" class="Bool (strict)"("Visible"=w1951) -> ()  [unwired: 2 in, 2 out]
            n1609 = property on="Port 3" class="Bool (strict)"("Visible"=w1951) -> ()  [unwired: 2 in, 2 out]
          }
        }
        n1610 = Wait (ms)(milliseconds to wait=u32 40) -> ()  [unwired: 1 out]
        n1611 = case shown="True" w1936 {
          tunnel: [w1948 errorcluster {"status"=TRUE, "code"=0, "source"="Init"} ("error out")] -> w1937
          tunnel: w1940 -> [w1948 _]
          frame False {
          }
          frame True {
          }
        }
        n1612 = case shown="Error" w1937 {
          selector: w1937 -> [w1958 w1976]
          tunnel: [w1961 w1980] -> w1947
          tunnel: [w1960 w1974] -> w1946
          tunnel: w1938 -> [w1959 w1978]
          frame No Error {
            n1613 = property class="Instr"(reference=w1959, error in=w1958) -> (reference out=w1956:refnum<visa-resource-name>, error out=w1957:errorcluster, "Serial Settings:Number of Bytes at Serial Port"=w1953:u32)
            n1614 = Greater?(x=w1953, y=u32 5) -> (0:w1952:bool)
            n1615 = Not(x=w1952) -> (.not. x?=→"Port 1a":bool)
            n1616 = while {
              tunnel: [w1969] -> w1960
              tunnel: [w1968] -> w1961
              tunnel: w1957 -> [w1967]
              tunnel: w1956 -> [w1966]
              stop <- TRUE stop-if-true
              n1617 = property class="Instr" props=["Serial Settings:Number of Bytes at Serial Port"](reference=w1966, error in=w1967) -> (reference out=w1971:refnum<visa-resource-name>, error out=w1970:errorcluster)  [unwired: 1 out]
              n1618 = VISA Read(VISA resource name=w1971, byte count=u32 50, error in (no error)=w1970) -> (VISA resource name out=w1968:refnum<visa-resource-name>, read buffer=w1963:string, error out=w1969:errorcluster)  [unwired: 1 out]
              n1619 = Wait (ms)(milliseconds to wait=u32 5) -> ()  [unwired: 1 out]
            }
          }
          frame Error {
            w1986 = u16 0 items=["None", "XON/XOFF", "RTS/CTS", "XON/XOFF & RTS/CTS", "DTR/DSR", "XON/XOFF & DTR/DSR"] ("flow control (0:none)  2")
            w1984 = u16 10 items=["1.0"=10, "1.5"=15, "2.0"=20] ("stop bits 2")
            w1982 = u16 0 items=["None", "Odd", "Even", "Mark", "Space"] ("parity 2")
            w1983 = u32 10000  # timeout (10sec)
            n1620 = VISA Close(VISA resource name=w1978, error in (no error)=w1976) -> (error out=w1979:errorcluster)
            n1621 = local write "Port 1a"(FALSE ("Port 1a")) -> ()
            n1622 = local read "Com Port 1"() -> (w1973:refnum<visa-resource-name>)
            n1623 = call <vilib>:"Clear Errors.vi"("error in (no error)"=w1979) -> ("error out"=w1977:errorcluster)  [unwired: 5 in, 1 out]
            n1624 = call-poly "VISA Configure Serial Port"("VISA resource name"=w1973, "timeout (10sec)"=w1983, "baud rate (9600)"=u32 250000 ("baud rate  2"), "data bits (8)"=u16 8 ("data bits  2"), "parity (0:none)"=w1982, "error in (no error)"=w1977, "stop bits (10: 1 bit)"=w1984, "flow control (0:none)"=w1986) -> ("VISA resource name out"=w1987:refnum<visa-resource-name>, "error out"=w1988:errorcluster)  [unwired: 6 in]
            n1625 = flat-sequence {
              tunnel: w1987 -> [w1990]
              tunnel: w1988 -> [w1989]
              tunnel: [w1990] -> w1980
              tunnel: [w1989] -> w1974
              frame #0 {
                n1626 = Wait (ms)(milliseconds to wait=u32 50) -> ()  [unwired: 1 out]
              }
            }
            "Residual Uno" <- ""
          }
        }
        n1627 = local read "Quit"() -> (w1935:bool)
        "Error Uno" <- w1940
      }
      n1628 = VISA Close(VISA resource name=w1933, error in (no error)=w1932) -> (error out=w1930:errorcluster)
      n1629 = call <vilib>:"Clear Errors.vi"("error in (no error)"=w1930) -> ()  [unwired: 5 in, 2 out]
    }
    frame Enabled {
    }
  }
  n1630 = while {
    stop <- w2001 stop-if-true
    # "V0OLTAGE TO STROKE (peice vise calibration)"
    n1631 = local read "LVDT MIN"() -> (w1993:dbl)
    n1632 = local read "LVDT Peak"() -> (w1992:dbl)
    n1633 = Wait (ms)(milliseconds to wait=u32 10) -> ()  [unwired: 1 out]
    n1634 = formula code="// Dynamic Parameterized Linear Interpolation Node\n// Inputs: vpp_val, voltages (Array), distances (Array)\n// Outputs: stroke\n\nint i = 0;\nint segments = 11; // 12 points make 11 interpolation segments\n\n// 1. Lower Boundary Clamp\nif (vpp_val <= voltages[0]) {\n    stroke = distances[0];\n}\n// 2. Upper Boundary Clamp\nelse if (vpp_val >= voltages[segments]) {\n    stroke = distances[segments];\n}\n// 3. Dynamic Segment Search Loop\nelse {\n    stroke = distances[0]; // Fallback baseline\n    for (i = 0; i < segments; i++) {\n        if (vpp_val >= voltages[i] && vpp_val <= voltages[i+1]) {\n            // Standard linear interpolation formula using array lookups\n            stroke = distances[i] + (vpp_val - voltages[i]) * (distances[i+1] - distances[i]) / (voltages[i+1] - voltages[i]);\n            break; // Segment found, safely exit the loop\n        }\n    }\n}"("vpp_val"=w1992, "voltages"="calibration values", "distances"="STROKE") -> ("stroke"=→"LVDT STROKE":dbl)
    n1635 = local read "Calibration Tare Value"() -> (w1997:dbl)
    n1636 = local read "Calibration Tare"() -> (w1995:bool)
    n1637 = Subtract(x=w1993, y=w1997) -> (x-y=→"LVDT STROKE  Calibration":dbl)
    n1638 = case shown="True" w1995 {
      selector: w1995 -> [_ w2003]
      tunnel: w1993 -> [_ w2004]
      frame False {
      }
      frame True {
        n1639 = Not(x=w2003) -> (.not. x?=w2002:bool)
        n1640 = local write "Calibration Tare"(w2002) -> ()
        "Calibration Tare Value" <- w2004
      }
    }
    n1641 = local read "Quit"() -> (w2001:bool)
  }
  n1642 = while {
    stop <- w2027 stop-if-true
    n1643 = local read "Due read"() -> (w2025:string)
    n1644 = call <vilib>:"High Resolution Polling Wait.vi"("seconds to wait"=0.02) -> ()  [unwired: 10 in, 1 out]
    n1645 = local read "Frictioin Force Raw"() -> (w2007:dbl)
    n1646 = Spreadsheet String To Array(delimiter (Tab)=";", format string="", spreadsheet string=w2025, array type (2D Dbl)=string[] []) -> (array=w2022:string[])
    n1647 = Fract/Exp String To Number(string=w2022) -> (number=w2021:dbl[])  [unwired: 3 in, 1 out]
    n1648 = call <vilib>:"Median Filter PtByPt.vi"("rank"=2, "x"=w2007) -> ("Filtered x"=→"Friction":dbl)  [unwired: 2 in, 1 out]
    n1649 = Index Array(array=w2021) -> (element #1=→"Sample Temperature":dbl, element #2=→"Target Sample Temperature":dbl, element #3=→"Current Duty Cycle":dbl, element #4=→"Ambient Temperature":dbl, element #5=→"Dac Status":dbl, element #6=→"Vpp":dbl, element #7=→"Active Error Code":dbl, element #8=→"Kp":dbl, element #9=→"Ki":dbl, element #10=→"Kd":dbl, element #11=→"SampleRaw":dbl, element #12=→"AmbRaw":dbl)  [unwired: 12 in]
    n1650 = local read "Quit"() -> (w2027:bool)
  }
  n1651 = while {
    shift-right: [w2041] -> w41
    shift-left: _ -> [w2033]
    shift-right: [w2028] -> w40
    shift-left: errorcluster {"status"=FALSE, "code"=0, "source"="Init"} ("error out") -> [w2035]
    tunnel: [w2030] -> w44
    tunnel: [w2040] -> _
    i -> [w2040]
    stop <- w2030 stop-if-true
    n1652 = local read "Com Port 2"() -> (w2034:refnum<visa-resource-name>)
    n1653 = local read "Port 2a"() -> (w2036:bool)
    n1654 = Unbundle(w2035) -> ("status"=→"Port 4":bool)  [unwired: 2 out]
    n1655 = call <vilib>:"High Resolution Polling Wait.vi"("seconds to wait"=0.02) -> ()  [unwired: 10 in, 1 out]
    n1656 = local read "Port 4"() -> (w2037:bool)
    n1657 = Not Equal?(x=w2034, y=w2033) -> (x != y?=w2032:bool)
    n1658 = Or(x=w2037, y=w2036) -> (x .or. y?=w2039:bool)
    n1659 = case shown="False" w2039 {
      frame False {
        w2044 = TRUE ("Visible")
        n1660 = property on="Port 2a" class="Bool (strict)"("Visible"=w2044) -> ()  [unwired: 2 in, 2 out]
        n1661 = property on="Port 4" class="Bool (strict)"("Visible"=w2044) -> ()  [unwired: 2 in, 2 out]
      }
      frame True {
        w2045 = TRUE ("Visible")
        n1662 = property on="Port 2a" class="Bool (strict)"("Visible"=w2045) -> ()  [unwired: 2 in, 2 out]
        n1663 = property on="Port 4" class="Bool (strict)"("Visible"=w2045) -> ()  [unwired: 2 in, 2 out]
      }
    }
    n1664 = case shown="True" w2032 {
      tunnel: [w2042 errorcluster {"status"=TRUE, "code"=0, "source"="Init"} ("error out")] -> w2031
      tunnel: w2035 -> [w2042 _]
      frame False {
      }
      frame True {
      }
    }
    n1665 = case shown="No Error" w2031 {
      selector: w2031 -> [w2058 w2089]
      tunnel: [w2051 w2094] -> w2041
      tunnel: [w2059 w2087] -> w2028
      tunnel: w2033 -> [w2060 w2092]
      frame No Error {
        n1666 = property class="Instr" props=["Serial Settings:Number of Bytes at Serial Port"](reference=w2060, error in=w2058) -> (reference out=w2052:refnum<visa-resource-name>, error out=w2057:errorcluster)  [unwired: 1 out]
        n1667 = while {
          tunnel: [w2068] -> w2053
          tunnel: [w2067] -> w2054
          tunnel: w2057 -> [w2066]
          tunnel: w2052 -> [w2065]
          tunnel: [w2064] -> _
          i -> [w2064]
          stop <- TRUE stop-if-true
          n1668 = property class="Instr" props=["Serial Settings:Number of Bytes at Serial Port"](reference=w2065, error in=w2066) -> (reference out=w2070:refnum<visa-resource-name>, error out=w2069:errorcluster)  [unwired: 1 out]
          n1669 = VISA Read(VISA resource name=w2070, byte count=u32 1000, error in (no error)=w2069) -> (VISA resource name out=w2067:refnum<visa-resource-name>, read buffer=→"Due read":string, error out=w2068:errorcluster)  [unwired: 1 out]
        }
        n1670 = local read "Due Write"() -> (w2050:string)
        n1671 = call <vilib>:"Trim Whitespace.vi"("string"=w2050) -> ("trimmed string"=w2049:string)  [unwired: 1 in]
        n1672 = Not Equal?(x=w2049, y="") -> (x != y?=w2055:bool)
        n1673 = VISA Flush I/O Buffer(VISA resource name=w2054) -> (VISA resource name out=w2047:refnum<visa-resource-name>, error out=→"error out 10":errorcluster)  [unwired: 2 in]
        n1674 = case shown="True" w2055 {
          tunnel: w2047 -> [w2072 w2077]
          tunnel: [w2072 w2081] -> w2051
          tunnel: w2053 -> [w2071 w2076]
          tunnel: [w2071 w2079] -> w2059
          tunnel: w2049 -> [_ w2075]
          tunnel: [_ w2078] -> _
          frame False {
            # "DATA  WRITE LOOP"
          }
          frame True {
            n1675 = Concatenate Strings(w2075, "\r\n") -> (w2074:string)
            n1676 = VISA Write(VISA resource name=w2077, write buffer=w2074, error in (no error)=w2076) -> (VISA resource name out=w2081:refnum<visa-resource-name>, return count=w2078:u32, error out=w2080:errorcluster)
            n1677 = flat-sequence {
              tunnel: w2080 -> [w2083]
              tunnel: [w2083] -> w2079
              frame #0 {
                n1678 = local write "Due Write"("" ("Command")) -> ()
                n1679 = Wait (ms)(milliseconds to wait=u32 5) -> ()  [unwired: 1 out]
              }
            }
          }
        }
        "Port 2a" <- TRUE ("Port 2a")
      }
      frame Error {
        w2100 = u16 0 items=["None", "XON/XOFF", "RTS/CTS", "XON/XOFF & RTS/CTS", "DTR/DSR", "XON/XOFF & DTR/DSR"] ("flow control (0:none)  2")
        w2098 = u16 10 items=["1.0"=10, "1.5"=15, "2.0"=20] ("stop bits 2")
        w2096 = u16 0 items=["None", "Odd", "Even", "Mark", "Space"] ("parity 2")
        w2097 = u32 10000  # timeout (10sec)
        n1680 = VISA Clear(VISA resource name=w2092, error in (no error)=w2089) -> (VISA resource name out=w2091:refnum<visa-resource-name>, error out=w2090:errorcluster)